vi "Main.vi"() -> ()   [LabVIEW 2018] (continued)
        n137 = Index Array(array=w350, index=2) -> (element=w360:cluster{"X":dbl[], "Y":dbl[]})
        n138 = Index Array(array=w350, index=3) -> (element=w359:cluster{"X":dbl[], "Y":dbl[]})
        n139 = Index Array(array=w350, index=0) -> (element=w362:cluster{"X":dbl[], "Y":dbl[]})
        n140 = Index Array(array=w350, index=1) -> (element=w361:cluster{"X":dbl[], "Y":dbl[]})
        n141 = Unbundle By Name(w359) -> ("Y"=w354:dbl[])
        n142 = Unbundle(w362) -> ("X"=w358:dbl[], "Y"=w357:dbl[])
        n143 = Unbundle By Name(w361) -> ("Y"=w356:dbl[])
        n144 = Unbundle By Name(w360) -> ("Y"=w355:dbl[])
        n145 = Transpose 2D Array(2D array=w371) -> (transposed array=w370:dbl[][])
        n146 = Build Array(w358, w357, w356, w355, w354) -> (w353:dbl[][])
        n147 = Transpose 2D Array(2D array=w353) -> (transposed array=w352:dbl[][])
        n148 = call "Save2CSV.vi"("Time Stamp?"=FALSE, "File Name"=w342, "error in"=w369, "Data Name"="Raw" ("string"), "Data 2D Array"=w370, "Parent Directory"=w364) -> ("error out"=w365:errorcluster)  [unwired: 4 in, 1 out]
        n149 = call "Save2CSV.vi"("Time Stamp?"=FALSE, "File Name"=w342, "error in"=w365, "Data Name"="Phase" ("string"), "Data 2D Array"=w352, "Parent Directory"=w364) -> ("error out"=w351:errorcluster)  [unwired: 4 in, 1 out]
      }
      event "Save #1": Value Change {
        n150 = event-data() -> ()  [unwired: 1 in, 1 out]
        n151 = local read "Wavelength (nm)"() -> (w393:string)
        n152 = local write "Wavelength #1"(w393) -> ()
        "[M/B]#1" <- "[M/B]"
        "Calibrated Bias #1" <- "Calibrated Bias (V)"
        "[O_B] #1" <- "[O_B]"
        "[d13]#1" <- "[d13]"
        "[d24]#1" <- "[d24]"
      }
      event "Load #1": Value Change {
        n153 = event-data() -> ()  [unwired: 1 in, 1 out]
        n154 = local read "[O_B] #1"() -> (w401:dbl)
        n155 = local read "[d13]#1"() -> (w397:dbl)
        n156 = local read "[d24]#1"() -> (w396:dbl)
        n157 = local read "Calibrated Bias #1"() -> (w403:dbl[])
        n158 = local read "[M/B]#1"() -> (w402:dbl)
        n159 = local write "[O_B]"(w401) -> ()
        n160 = local write "Calibrated Bias (V)"(w403) -> ()
        n161 = local write "Wavelength (nm)"("Wavelength #1") -> ()
        n162 = local write "[M/B]"(w402) -> ()
        n163 = local write "[d13]"(w397) -> ()
        n164 = local write "[d24]"(w396) -> ()
      }
      event "Save #2": Value Change {
        n165 = event-data() -> ()  [unwired: 1 in, 1 out]
        n166 = local read "[d13]"() -> (→"[d13]#2":dbl)
        n167 = local read "[O_B]"() -> (→"[O_B]#2":dbl)
        n168 = local read "[d24]"() -> (→"[d24]#2":dbl)
        n169 = local read "Calibrated Bias (V)"() -> (→"Calibrated Bias #2":dbl[])
        n170 = local read "Wavelength (nm)"() -> (w410:string)
        n171 = local read "[M/B]"() -> (→"[M/B]#2":dbl)
        n172 = local write "Wavelength #2"(w410) -> ()
      }
      event "Load #2": Value Change {
        n173 = event-data() -> ()  [unwired: 1 in, 1 out]
        n174 = local read "[O_B]#2"() -> (w421:dbl)
        n175 = local read "[d13]#2"() -> (w417:dbl)
        n176 = local read "Calibrated Bias #2"() -> (w425:dbl[])
        n177 = local read "[d24]#2"() -> (w416:dbl)
        n178 = local read "[M/B]#2"() -> (w424:dbl)
        n179 = local write "[O_B]"(w421) -> ()
        n180 = local write "Wavelength (nm)"("Wavelength #2") -> ()
        n181 = local write "Calibrated Bias (V)"(w425) -> ()
        n182 = local write "[M/B]"(w424) -> ()
        n183 = local write "[d24]"(w416) -> ()
        n184 = local write "[d13]"(w417) -> ()
      }
      event "Save #3": Value Change {
        n185 = event-data() -> ()  [unwired: 1 in, 1 out]
        n186 = local read "[O_B]"() -> (→"[O_B]#3":dbl)
        n187 = local read "[d24]"() -> (→"[d24]#3":dbl)
        n188 = local read "[d13]"() -> (→"[d13]#3":dbl)
        n189 = local read "Calibrated Bias (V)"() -> (→"Calibrated Bias #3":dbl[])
        n190 = local read "Wavelength (nm)"() -> (w430:string)
        n191 = local read "[M/B]"() -> (→"[M/B]#3":dbl)
        n192 = local write "Wavelength #3"(w430) -> ()
      }
      event "Load #3": Value Change {
        n193 = event-data() -> ()  [unwired: 1 in, 1 out]
        n194 = local read "[O_B]#3"() -> (w441:dbl)
        n195 = local read "[d13]#3"() -> (w437:dbl)
        n196 = local read "[d24]#3"() -> (w436:dbl)
        n197 = local read "Calibrated Bias #3"() -> (w443:dbl[])
        n198 = local read "[M/B]#3"() -> (w442:dbl)
        n199 = local write "[O_B]"(w441) -> ()
        n200 = local write "Wavelength (nm)"("Wavelength #3") -> ()
        n201 = local write "Calibrated Bias (V)"(w443) -> ()
        n202 = local write "[M/B]"(w442) -> ()
        n203 = local write "[d13]"(w437) -> ()
        n204 = local write "[d24]"(w436) -> ()
      }
      event "Save #4": Value Change {
        n205 = event-data() -> ()  [unwired: 1 in, 1 out]
        n206 = local read "[d13]"() -> (→"[d13]#4":dbl)
        n207 = local read "[d24]"() -> (→"[d24]#4":dbl)
        n208 = local read "[O_B]"() -> (→"[O_B]#4":dbl)
        n209 = local read "Calibrated Bias (V)"() -> (→"Calibrated Bias #4":dbl[])
        n210 = local read "Wavelength (nm)"() -> (w450:string)
        n211 = local read "[M/B]"() -> (→"[M/B]#4":dbl)
        n212 = local write "Wavelength #4"(w450) -> ()
      }
      event "Load #4": Value Change {
        n213 = event-data() -> ()  [unwired: 1 in, 1 out]
        n214 = local read "[O_B]#4"() -> (w461:dbl)
        n215 = local read "[d13]#4"() -> (w457:dbl)
        n216 = local read "Calibrated Bias #4"() -> (w463:dbl[])
        n217 = local read "[d24]#4"() -> (w456:dbl)
        n218 = local read "[M/B]#4"() -> (w462:dbl)
        n219 = local write "[O_B]"(w461) -> ()
        n220 = local write "Wavelength (nm)"("Wavelength #4") -> ()
        n221 = local write "Calibrated Bias (V)"(w463) -> ()
        n222 = local write "[M/B]"(w462) -> ()
        n223 = local write "[d13]"(w457) -> ()
        n224 = local write "[d24]"(w456) -> ()
      }
      event "Fast Scan": Value Change {
        # "Repeat for Fast Scan"
        n225 = event-data() -> ()  [unwired: 1 in, 1 out]
        n226 = flat-sequence {
          tunnel: w482 -> [w489]
          tunnel: [w489] -> w478
          tunnel: [w488] -> w477
          tunnel: [w487] -> w476
          tunnel: w480 -> [w487]
          tunnel: [w486] -> w475
          tunnel: w479 -> [w486]
          tunnel: w474 -> [w484]
          tunnel: [w483] -> w473
          tunnel: w478 -> [w518]
          tunnel: [w518] -> w470
          tunnel: w477 -> [w517]
          tunnel: [w517] -> w469
          tunnel: w476 -> [w513]
          tunnel: w475 -> [w500]
          tunnel: [w510] -> w468
          tunnel: w473 -> [w509]
          tunnel: [w498] -> w466
          tunnel: [w546] -> w472
          tunnel: [w547] -> w481
          tunnel: w470 -> [w547]
          tunnel: w468 -> [w543]
          tunnel: w469 -> [w537]
          tunnel: w466 -> [w530]
          frame #0 {
            n227 = local read "Shutter"() -> (w485:bool)
            n228 = case shown="False" w485 {
              tunnel: w484 -> [w493 w495]
              tunnel: [w492 w495] -> w483
              frame False {
                n229 = local read "Shutter Line"() -> (w490:tag)
                n230 = call "ShutterControl.vi"("error in"=w493, "Shutter Line"=w490, "Shutter"=TRUE) -> ("error out"=w492:errorcluster, "Status Indicator"=w491:bool)  [unwired: 7 in]
                n231 = local write "Shutter"(w491) -> ()
              }
              frame True {
              }
            }
            n232 = Tick Count (ms)() -> (millisecond timer value=w488:u32)
          }
          frame #1 {
            w503 = T13."Fast Scan" ("Main Tab")
            n233 = local read "AOStartTrigger"() -> (w496:tag)
            n234 = local read "AIStartTrigger"() -> (w497:tag)
            n235 = call "DAQInit.vi"("AOStartTrigger"=w496, "AIStartTrigger"=w497, "Scan/Meas Parameters"="Fast Scan Parameters", "error in"=w509, "Functions"=w503, "Global Parameters"=w500, "DAQ Channels"=w513) -> ("error out"=w511:errorcluster, "Expected Time (s)"=→"Expected Frame Time (s)":dbl, "Tasks Out"=w515:T14)  [unwired: 2 in]
            n236 = call "ScanXY.vi"("Scan/Meas Parameters"="Fast Scan Parameters") -> ("XYcoordinates"=w504:dbl[][])  [unwired: 10 in]
            n237 = Unbundle By Name("Fast Scan Parameters") -> ("Pixel Size"=w508:dbl)
            n238 = case shown="True" "Single Pixel?" {
              tunnel: [w519 w520] -> w505
              tunnel: w504 -> [w519 w521]
              frame False {
              }
              frame True {
                n239 = Multiply(x=w521, y=0.0) -> (x*y=w520:dbl[][])
              }
            }
            n240 = To Long Integer(number=w508) -> (32bit integer=w507:i32)
            n241 = call "ImageFrame.vi"("Tasks In"=w515, "Functions"=w503, "error in"=w511, "XYcoordinates"=w505) -> ("Tasks Out"=w512:T14, "DC AI Channel Date"=w501:dbl[], "error out"=w514:errorcluster)  [unwired: 7 in, 2 out]
            n242 = call "Analysis.vi"("Functions"=w503, "Scan/Meas Parameters"="Fast Scan Parameters", "Global Parameters"=w500, "DC AI Channel Data"=w501) -> ("AI DC Data"=w498:dbl[])  [unwired: 2 in, 5 out]
            n243 = Reshape Array(w498, w507, w507) -> (→"Fast Scan Intensity Image":dbl[][])
            n244 = call "DAQClose.vi"("error in"=w514, "Functions"=w503, "Tasks In"=w512, "DAQ Channels"=w513) -> ("error out"=w510:errorcluster)  [unwired: 7 in]
          }
          frame #2 {
            n245 = local read "Simple Max Search"() -> (w533:bool)
            n246 = local read "Shutter Line"() -> (w523:tag)
            n247 = local read "Export Z Calibration"() -> (w524:bool)
            n248 = Tick Count (ms)() -> (millisecond timer value=w538:u32)
            n249 = call "ShutterControl.vi"("error in"=w543, "Shutter Line"=w523, "Shutter"=FALSE) -> ("error out"=w542:errorcluster, "Status Indicator"=w544:bool)  [unwired: 7 in]
            n250 = local read "Quadratic Search"() -> (w526:bool)
            n251 = local write "Shutter"(w544) -> ()
            n252 = call <vilib>:"Std Deviation and Variance.vi"("X"=w530) -> ("mean"=w525:dbl, "variance"=w531:dbl)  [unwired: 1 in, 1 out]
            "Mean Pixel Value" <- w525
            n253 = Subtract(x=w538, y=w537) -> (x-y=w540:u32)
            n254 = Square(x=w525) -> (x^2=w532:dbl)
            n255 = local read "SPGD"() -> (w534:bool)
            n256 = To Double Precision Float(number=w540) -> (double precision float=w541:dbl)
            n257 = Divide(x=w531, y=w532) -> (x/y=w527:dbl)
            "Normalized Variance" <- w527
            n258 = Divide(x=w541, y=1000.0) -> (x/y=→"Actual Scan Time (s)":dbl)
            n259 = Compound Arithmetic op=OR(w526, w534, w533, w524) -> (w535:bool)
            n260 = case shown="False" w535 {
              tunnel: [w563 w570] -> w546
              tunnel: w542 -> [w561 w570]
              frame False {
                n261 = local read "Fast Scan Progress"() -> (w557:dbl)
                n262 = Reciprocal(x="Fast Scan Frames") -> (1/x=w558:dbl)
                n263 = Multiply(x=100.0, y=w558) -> (x*y=w560:dbl)
                n264 = Add(x=w557, y=w560) -> (x+y=w553:dbl)
                "Fast Scan Progress" <- w553
                n265 = Greater Or Equal?(x=w553, y=100.0) -> (x >= y?=w554:bool)
                n266 = Compound Arithmetic op=OR(w554, "Stop Fast Scan") -> (w562:bool)
                n267 = case shown="True" w562 {
                  tunnel: w561 -> [w566 w567]
                  tunnel: [w565 w567] -> w563
                  frame False {
                    # "Continue Fast Scan"
                    n268 = property on="Fast Scan" class="Bool (strict)"(error in=w566, "Val(Sgnl)"=TRUE ("Value (Signaling)")) -> (error out=w565:errorcluster)  [unwired: 1 in, 1 out]
                  }
                  frame True {
                    w569 = FALSE ("Fast Scan")
                    # "Fast Scan Stops"
                    n269 = local write "Fast Scan Progress"(0.0 ("Fast Scan Progress")) -> ()
                    n270 = local write "Fast Scan"(w569) -> ()
                    n271 = local write "Stop Fast Scan"(w569) -> ()
                  }
                }
              }
              frame True {
              }
            }
            n272 = case shown="\"Mean Pixel Value\", Default" "Optimization Metric" {
              tunnel: [w548 w549 w550] -> w528
              tunnel: w525 -> [w548 _ w551]
              tunnel: w527 -> [_ w549 _]
              frame "Mean Pixel Value", Default {
              }
              frame "Normalized Variance" {
              }
              frame "Mean Squared Pixel Value" {
                n273 = Square Root(x=w551) -> (sqrt(x)=w550:dbl)
              }
            }
            "Metric Value" <- w528
          }
        }
      }
      event "Relax DM": Value Change {
        n274 = event-data() -> ()  [unwired: 1 in, 1 out]
        n275 = local read "Use DM?"() -> (w571:bool)
        n276 = case shown="True" w571 {
          tunnel: [w579 w583] -> w576
          tunnel: [w578 w582] -> w575
          tunnel: w573 -> [w579 w581]
          tunnel: w572 -> [w578 w580]
          frame False {
          }
          frame True {
            w591 = u32 0 items=["Mirror", "Arms", "Mirror + Arms"] ("Device Part (Mirror)")
            # "First Step"
            n277 = call "TLDFMX Relax.vi"("Reload (1)"=TRUE, "error in (no error)"=w580, "Is First Step (0)"=TRUE, "Device Part (Mirror)"=w591, "instrument handle"=w581) -> ("error out"=w587:errorcluster, "Relax Pattern Mirror (0)"=w586:dbl[], "instrument handle out"=w588:refnum<visa-resource-name>)  [unwired: 2 in, 2 out]
            n278 = call "TLDFM Set Segment Voltages.vi"("error in (no error)"=w587, "Segment Voltages"=w586, "instrument handle"=w588) -> ("error out"=w584:errorcluster, "instrument handle out"=w585:refnum<visa-resource-name>)  [unwired: 7 in]
            n279 = while {
              tunnel: w585 -> [w597]
              tunnel: w584 -> [w596]
              tunnel: [w593] -> w583
              tunnel: [w592] -> w582
              stop <- w594 stop-if-true
              w598 = u32 0 items=["Mirror", "Arms", "Mirror + Arms"] ("Device Part (Mirror)")
              # "Loop Until Remaining Relax Steps Are 0"
              n280 = call "TLDFMX Relax.vi"("Reload (1)"=TRUE, "error in (no error)"=w596, "Is First Step (0)"=FALSE, "Device Part (Mirror)"=w598, "instrument handle"=w597) -> ("error out"=w602:errorcluster, "Relax Pattern Mirror (0)"=w603:dbl[], "instrument handle out"=w601:refnum<visa-resource-name>, "Remaining Steps"=w595:i32)  [unwired: 2 in, 1 out]
              n281 = Less Or Equal To 0?(x=w595) -> (x <= 0?=w594:bool)
              n282 = call "TLDFM Set Segment Voltages.vi"("error in (no error)"=w602, "Segment Voltages"=w603, "instrument handle"=w601) -> ("error out"=w592:errorcluster, "instrument handle out"=w593:refnum<visa-resource-name>)  [unwired: 7 in]
            }
          }
        }
      }
      event "Reset Zernike": Value Change {
        n283 = event-data() -> ()  [unwired: 1 in, 1 out]
        n284 = local read "Use DM?"() -> (w604:bool)
        n285 = local write "Zernike Array"(dbl[] [0.0, 0.0, 0.0, 0.0, 0.0, 0.0, 0.0, 0.0, 0.0, 0.0, 0.0, 0.0] ("Zernike Array")) -> ()
        n286 = case shown="False" w604 {
          tunnel: w608 -> [w612 w616]
          tunnel: w607 -> [w611 w615]
          tunnel: [w612 w614] -> w606
          tunnel: [w611 w613] -> w605
          frame False {
          }
          frame True {
            n287 = call "TLDFMX Reset.vi"("error in (no error)"=w615, "instrument handle"=w616) -> ("error out"=w613:errorcluster, "instrument handle out"=w614:refnum<visa-resource-name>)  [unwired: 8 in]
          }
        }
      }
      event "Zernike Array", "Apply Zernike": Value Change {
        n288 = event-data() -> ()  [unwired: 1 in, 1 out]
        n289 = local read "Use DM?"() -> (w617:bool)
        n290 = case shown="True" w617 {
          tunnel: w623 -> [w624 w637]
          tunnel: w622 -> [w625 w635]
          tunnel: [w624 w631] -> w621
          tunnel: [w625 w630] -> w619
          frame False {
          }
          frame True {
            n291 = local read "Zernike Enable"() -> (w629:bool[])
            n292 = Boolean To (0,1)(Boolean=w629) -> (0, 1=w628:i16[])
            n293 = Multiply(x="Zernike Array", y=w628) -> (x*y=w626:dbl[])
            n294 = call "TLDFMX Calculate Zernike Pattern.vi"("error in (no error)"=w637, "Zernike Amplitudes"=w626, "Zernikes"=u32 4294967295, "instrument handle"=w635) -> ("error out"=w632:errorcluster, "Mirror Pattern"=w633:dbl[], "instrument handle out"=w634:refnum<visa-resource-name>)  [unwired: 5 in]
            n295 = call "TLDFM Set Segment Voltages.vi"("error in (no error)"=w632, "Segment Voltages"=w633, "instrument handle"=w634) -> ("error out"=w631:errorcluster, "instrument handle out"=w630:refnum<visa-resource-name>)  [unwired: 7 in]
          }
        }
      }
      event "Save Zernike": Value Change {
        w655 = "DM" ("section")
        n296 = event-data() -> ()  [unwired: 1 in, 1 out]
        n297 = Current VI's Path() -> (path=w639:path)
        n298 = Strip Path(path=w639) -> (stripped path=w638:path)  [unwired: 1 out]
        n299 = Build Path(base path=w638, name or relative path=path "config.ini" ("default name")) -> (appended path=w665:path)
        n300 = local read "Zernike Array"() -> (w649:dbl[])
        n301 = call <vilib>:"Open Config Data.vi"("error in (no error)"=w664, "create file if necessary (T)"=TRUE, "configuration file path"=w665) -> ("error out"=w663:errorcluster, "refnum"=w661:T15)  [unwired: 6 in, 1 out]
        n302 = Array To Spreadsheet String(delimiter (Tab)=",", array=w649, 3:"%#g" ("format string")) -> (spreadsheet string=w653:string)
        n303 = Search and Replace String(input string=w653, search string="\r\n") -> (result string=w648:string)  [unwired: 6 in, 3 out]
        n304 = call-poly <vilib>:"Write Key.vi"("section"=w655, "error in (no error)"=w663, "value"=w648, "key"="Zernike Array", "refnum"=w661) -> ("error out"=w657:errorcluster, "refnum out"=w659:T15)  [unwired: 4 in, 1 out]
        n305 = local read "Zernike Enable"() -> (w642:bool[])
        n306 = for {
          tunnel: w642 -> [w670] mode=indexing
          tunnel: [w669] -> w643 mode=indexing
          n307 = Select(t="TRUE", s=w670, f="FALSE") -> (s? t:f=w669:string)
        }
        n308 = Array To Spreadsheet String(delimiter (Tab)=",", array=w643, 3:"%s" ("format string")) -> (spreadsheet string=w647:string)
        n309 = Search and Replace String(input string=w647, search string="\r\n") -> (result string=w641:string)  [unwired: 6 in, 3 out]
        n310 = call-poly <vilib>:"Write Key.vi"("section"=w655, "error in (no error)"=w657, "value"=w641, "key"="Zernike Enable", "refnum"=w659) -> ("error out"=w656:errorcluster, "refnum out"=w658:T15)  [unwired: 4 in, 1 out]
        n311 = call <vilib>:"Close Config Data.vi"("error in (no error)"=w656, "refnum"=w658) -> ("error out"=w662:errorcluster)  [unwired: 8 in, 1 out]
      }
      event "Load Zernike": Value Change {
        n312 = event-data() -> ()  [unwired: 1 in, 1 out]
        n313 = Current VI's Path() -> (path=w680:path)
        n314 = Strip Path(path=w680) -> (stripped path=w679:path)  [unwired: 1 out]
        n315 = Build Path(base path=w679, name or relative path=path "config.ini" ("default name")) -> (appended path=w677:path)
        n316 = call <vilib>:"Check if File or Folder Exists.vi"("error in (no error)"=w676, "path"=w677) -> ("error out"=w675:errorcluster, "file or folder exists?"=w673:bool, "dup path"=w674:path)  [unwired: 7 in]
        n317 = case shown="True" w673 {
          tunnel: [w684 w708] -> w678
          tunnel: w675 -> [w684 w686]
          tunnel: w674 -> [_ w685]
          frame False {
          }
          frame True {
            w688 = "DM" ("section")
            n318 = call <vilib>:"Open Config Data.vi"("error in (no error)"=w686, "create file if necessary (T)"=FALSE, "configuration file path"=w685) -> ("error out"=w701:errorcluster, "refnum"=w702:T15)  [unwired: 6 in, 1 out]
            n319 = call-poly <vilib>:"Read Key.vi"("section"=w688, "error in (no error)"=w701, "key"="Zernike Array", "refnum"=w702) -> ("error out"=w693:errorcluster, "value"=w704:string, "refnum out"=w691:T15)  [unwired: 4 in, 1 out]
            n320 = Spreadsheet String To Array(delimiter (Tab)=",", format string="%s", spreadsheet string=w704, array type (2D Dbl)=dbl[] []) -> (array=w700:dbl[])
            n321 = local write "Zernike Array"(w700) -> ()
            n322 = call-poly <vilib>:"Read Key.vi"("section"=w688, "error in (no error)"=w693, "key"="Zernike Enable", "refnum"=w691) -> ("error out"=w692:errorcluster, "value"=w696:string, "refnum out"=w690:T15)  [unwired: 4 in, 1 out]
            n323 = Spreadsheet String To Array(delimiter (Tab)=",", format string="%s", spreadsheet string=w696, array type (2D Dbl)=string[] []) -> (array=w694:string[])
            n324 = for {
              tunnel: "TRUE" -> [w712]
              tunnel: w694 -> [w711] mode=indexing
              tunnel: [w710] -> w687 mode=indexing
              n325 = Equal?(x=w711, y=w712) -> (x = y?=w710:bool)
            }
            n326 = local write "Zernike Enable"(w687) -> ()
            n327 = call <vilib>:"Close Config Data.vi"("error in (no error)"=w692, "refnum"=w690) -> ("error out"=w708:errorcluster)  [unwired: 8 in, 1 out]
          }
        }
      }
      event "Quadratic Search": Value Change {
        n328 = event-data() -> ()  [unwired: 1 in, 1 out]
        n329 = while {
          tunnel: [w814] -> w720
          tunnel: [w816] -> w724
          stop <- w817 stop-if-true
          n330 = local read "Zernike Enable"() -> (w815:bool[])
          n331 = local read "Current Z Idx"() -> (w820:i32)
          n332 = Index Array(array=w815, index=w820) -> (element=w821:bool)
          n333 = Array Size(array=w815) -> (size(s)=w819:i32)
          n334 = case shown="True" w821 {
            tunnel: w820 -> [w825 w827]
            tunnel: [w824 w827] -> w814
            tunnel: [FALSE ("2D Time-Lapse Measure") TRUE ("2D Time-Lapse Measure")] -> w818
            frame False {
              n335 = local write "Z Direction"(TRUE ("Zernike Dir")) -> ()
              n336 = Increment(x=w825) -> (x+1=w824:i32)
            }
            frame True {
            }
          }
          n337 = Greater?(x=w814, y=w819) -> (0:w816:bool)
          n338 = local write "Current Z Idx"(w814) -> ()
          n339 = Compound Arithmetic op=OR(w818, w816) -> (w817:bool)
        }
        n340 = local read "Current Iteration"() -> (w713:sgl)
        n341 = local read "Quadratic Calc"() -> (w716:bool)
        n342 = case shown="False" w716 {
          tunnel: w715 -> [w727 w731]
          tunnel: [w727 w731] -> w714
          tunnel: w713 -> [w726 _]
          frame False {
            n343 = Equal To 0?(x=w726) -> (x = 0?=w725:bool)
            n344 = case shown="True" w725 {
              frame False {
              }
              frame True {
                n345 = local read "Zernike Array"() -> (w728:dbl[])
                n346 = local write "Optimal Z Idx"(0 ("Optimal Z Idx")) -> ()
                n347 = local write "Optimal Zernike"(w728) -> ()
              }
            }
          }
          frame True {
            n348 = local read "Bias Amplitude"() -> (w740:dbl)
            n349 = local read "Optimal Zernike"() -> (w734:dbl[])
            n350 = local read "Initial Metric"() -> (w742:dbl)
            n351 = local read "Metric Value"() -> (w741:dbl)
            n352 = local read "Last Metric"() -> (w743:dbl)
            n353 = local read "Optimal Z Idx"() -> (w730:i32)
            n354 = call "QuadraticOptimization.vi"("Bias Amplitude"=w740, "Neg Metric"=w741, "Initial Metric"=w742, "Pos Metric"=w743) -> ("Opt Variable (compared to 0)"=w732:dbl)  [unwired: 7 in]
            n355 = Index Array(array=w734, index=w730) -> (element=w736:dbl)
            n356 = Add(x=w736, y=w732) -> (x+y=w737:dbl)
            n357 = In Range and Coerce(upper limit=1.0 ("y"), x=w737, lower limit=-1.0 ("y")) -> (coerced(x)=w735:dbl)  [unwired: 1 out]
            n358 = Replace Array Subset(array=w734, new element=w735, index=w730) -> (→"Optimal Zernike":dbl[])
          }
        }
        n359 = local read "Stop AO Algorithm"() -> (w723:bool)
        n360 = Compound Arithmetic op=OR(w724, w723) -> (w722:bool)
        n361 = case shown="False" w722 {
          tunnel: w714 -> [w755 w803]
          tunnel: [w750 w802] -> w721
          tunnel: w718 -> [w756 w800]
          tunnel: [w757 w801] -> w717
          tunnel: w713 -> [w747 _]
          tunnel: w720 -> [w752 _]
          frame False {
            w749 = TRUE ("Value (Signaling)")
            n362 = Equal To 0?(x=w747) -> (x = 0?=w753:bool)
            n363 = case shown="False" w753 {
              tunnel: [w776 w793] -> w748
              tunnel: [w778 w794] -> w744
              tunnel: w752 -> [w764 _]
              frame False {
                n364 = local read "Initial Zernike"() -> (w765:dbl[])
                n365 = local read "Z Direction"() -> (w775:bool)
                n366 = case shown="False" w775 {
                  tunnel: "Bias Amplitude" -> [w786 w791]
                  tunnel: [w785 w791] -> w773
                  tunnel: [FALSE ("Zernike Dir") TRUE ("Zernike Dir")] -> w768
                  tunnel: w764 -> [w782 _]
                  frame False {
                    # "Negative Bias"
                    n367 = Multiply(x=w786, y=-1.0) -> (x*y=w785:dbl)
                    "Quadratic Calc" <- TRUE ("Quadratic Calc")
                    "Optimal Z Idx" <- w782
                  }
                  frame True {
                    # "Positive Bias"
                    n368 = local write "Quadratic Calc"(FALSE ("Zernike Dir")) -> ()
                    n369 = local write "Z Direction"(FALSE ("Zernike Dir")) -> ()
                  }
                }
                n370 = Index Array(array=w765, index=w764) -> (element=w777:dbl)
                n371 = Add(x=w777, y=w773) -> (x+y=w770:dbl)
                n372 = In Range and Coerce(upper limit=1.0 ("y"), x=w770, lower limit=-1.0 ("y")) -> (coerced(x)=w769:dbl, In Range?=w767:bool)
                n373 = Compound Arithmetic op=AND(w767, w768) -> (w766:bool)
                n374 = case shown="False" w766 {
                  tunnel: w764 -> [w780 _]
                  frame False {
                    n375 = Increment(x=w780) -> (x+1=w781:i32)
                    n376 = local write "Z Direction"(TRUE ("Zernike Dir")) -> ()
                    n377 = local write "Current Z Idx"(w781) -> ()
                  }
                  frame True {
                  }
                }
                n378 = local read "Metric Value"() -> (w778:dbl)
                n379 = Replace Array Subset(array=w765, new element=w769, index=w764) -> (w776:dbl[])
              }
              frame True {
                n380 = local read "Zernike Array"() -> (w793:dbl[])
                "Initial Zernike" <- w793
                n381 = local read "Last Metric"() -> (w794:dbl)
                n382 = local write "Quadratic Calc"(FALSE ("Zernike Dir")) -> ()
              }
            }
            n383 = Increment(x=w747) -> (x+1=w754:sgl)
            n384 = local write "Current Iteration"(w754) -> ()
            n385 = call "TLDFMX Calculate Zernike Pattern.vi"("error in (no error)"=w755, "Zernike Amplitudes"=w748, "Zernikes"=u32 4294967295, "instrument handle"=w756) -> ("error out"=w759:errorcluster, "Mirror Pattern"=w760:dbl[], "instrument handle out"=w761:refnum<visa-resource-name>)  [unwired: 5 in]
            n386 = call "TLDFM Set Segment Voltages.vi"("error in (no error)"=w759, "Segment Voltages"=w760, "instrument handle"=w761) -> ("error out"=w758:errorcluster, "instrument handle out"=w757:refnum<visa-resource-name>)  [unwired: 7 in]
            n387 = Equal?(x=w747, y=sgl 1.0) -> (x = y?=w745:bool)
            n388 = property on="Fast Scan" class="Bool (strict)"(error in=w758, "Val(Sgnl)"=w749) -> (error out=w751:errorcluster)  [unwired: 1 in, 1 out]
            n389 = case shown="True" w745 {
              tunnel: w744 -> [_ w763]
              frame False {
              }
              frame True {
                "Initial Metric" <- w763
              }
            }
            n390 = local write "Zernike Array"(w748) -> ()
            n391 = property on="Quadratic Search" class="Bool (strict)"(error in=w751, "Val(Sgnl)"=w749) -> (error out=w750:errorcluster)  [unwired: 1 in, 1 out]
            n392 = local write "Last Metric"(w744) -> ()
          }
          frame True {
            w813 = FALSE ("2D Time-Lapse Measure")
            n393 = local read "Zernike Enable"() -> (w799:bool[])
            n394 = local read "Optimal Zernike"() -> (w797:dbl[])
            n395 = Boolean To (0,1)(Boolean=w799) -> (0, 1=w798:i16[])
            n396 = Multiply(x=w797, y=w798) -> (x*y=w796:dbl[])
            n397 = call "TLDFMX Calculate Zernike Pattern.vi"("error in (no error)"=w803, "Zernike Amplitudes"=w796, "Zernikes"=u32 4294967295, "instrument handle"=w800) -> ("error out"=w804:errorcluster, "Mirror Pattern"=w805:dbl[], "instrument handle out"=w806:refnum<visa-resource-name>)  [unwired: 5 in]
            n398 = local write "Zernike Array"(w797) -> ()
            n399 = call "TLDFM Set Segment Voltages.vi"("error in (no error)"=w804, "Segment Voltages"=w805, "instrument handle"=w806) -> ("error out"=w802:errorcluster, "instrument handle out"=w801:refnum<visa-resource-name>)  [unwired: 7 in]
            n400 = local write "Optimal Z Idx"(0 ("Optimal Z Idx")) -> ()
            n401 = local write "Quadratic Calc"(FALSE ("Zernike Dir")) -> ()
            n402 = local write "Current Iteration"(sgl 0.0 ("Current Step")) -> ()
            n403 = local write "Quadratic Search"(w813) -> ()
            n404 = local write "Z Direction"(TRUE ("Zernike Dir")) -> ()
            n405 = local write "Fast Scan Progress"(0.0 ("Fast Scan Progress")) -> ()
            n406 = local write "Current Z Idx"(0 ("Curr Zernike Idx")) -> ()
            n407 = local write "Fast Scan"(w813) -> ()
            n408 = local write "Stop Fast Scan"(w813) -> ()
            n409 = local write "Stop AO Algorithm"(w813) -> ()
          }
        }
      }
      event "Simple Max Search": Value Change {
        n410 = event-data() -> ()  [unwired: 1 in, 1 out]
        n411 = while {
          tunnel: [w838] -> w828
          tunnel: [w840] -> w830
          stop <- w841 stop-if-true
          n412 = local read "Zernike Enable"() -> (w839:bool[])
          n413 = local read "Current Z Idx"() -> (w844:i32)
          n414 = Index Array(array=w839, index=w844) -> (element=w845:bool)
          n415 = Array Size(array=w839) -> (size(s)=w843:i32)
          n416 = case shown="False" w845 {
            tunnel: w844 -> [w849 w851]
            tunnel: [w848 w851] -> w838
            tunnel: [FALSE ("2D Time-Lapse Measure") TRUE ("2D Time-Lapse Measure")] -> w842
            frame False {
              n417 = local write "Z Direction"(TRUE ("Zernike Dir")) -> ()
              n418 = Increment(x=w849) -> (x+1=w848:i32)
            }
            frame True {
            }
          }
          n419 = Greater?(x=w838, y=w843) -> (0:w840:bool)
          n420 = local write "Current Z Idx"(w838) -> ()
          n421 = Compound Arithmetic op=OR(w842, w840) -> (w841:bool)
        }
        n422 = local read "Stop AO Algorithm"() -> (w832:bool)
        n423 = local read "Current Iteration"() -> (w829:sgl)
        n424 = Compound Arithmetic op=OR(w830, w832) -> (w831:bool)
        n425 = case shown="False" w831 {
          tunnel: w836 -> [w852 w909]
          tunnel: w835 -> [w853 w910]
          tunnel: [w867 w910] -> w834
          tunnel: [w864 w909] -> w833
          tunnel: w829 -> [w856 _]
          tunnel: w828 -> [w857 _]
          frame False {
            w863 = TRUE ("Value (Signaling)")
            n426 = Equal To 0?(x=w856) -> (x = 0?=w862:bool)
            n427 = Increment(x=w856) -> (x+1=w855:sgl)
            n428 = case shown="True" w862 {
              tunnel: [w879 w905] -> w859
              tunnel: w857 -> [w874 _]
              tunnel: [w872 w904] -> w854
              frame False {
                n429 = local read "Metric Value"() -> (w872:dbl)
                n430 = local read "Zernike Array"() -> (w881:dbl[])
                n431 = local read "Last Metric"() -> (w873:dbl)
                n432 = local read "Z Direction"() -> (w875:bool)
                n433 = Greater?(x=w872, y=w873) -> (0:w878:bool)
                n434 = Index Array(array=w881, index=w874) -> (element=w882:dbl)
                n435 = case shown="True" w875 {
                  tunnel: w878 -> [w886 w897]
                  tunnel: "Step Size" -> [w885 w896]
                  tunnel: [w884 w895] -> w876
                  tunnel: w874 -> [w883 _]
                  frame False {
                    # "Decreasing Zernike Coefficient"
                    n436 = case shown="True" w886 {
                      tunnel: w885 -> [w890 w892]
                      tunnel: [w890 w891] -> w884
                      tunnel: w883 -> [w888 _]
                      frame False {
                        n437 = Increment(x=w888) -> (x+1=w889:i32)
                        n438 = local write "Z Direction"(TRUE ("Zernike Dir")) -> ()
                        n439 = local write "Current Z Idx"(w889) -> ()
                      }
                      frame True {
                        n440 = local write "Z Direction"(FALSE ("Zernike Dir")) -> ()
                        n441 = Multiply(x=w892, y=-1.0) -> (x*y=w891:dbl)
                      }
                    }
                  }
                  frame True {
                    # "Increasing Zernike Coefficient"
                    n442 = case shown="False" w897 {
                      tunnel: w896 -> [w901 w903]
                      tunnel: [w900 w903] -> w895
                      frame False {
                        n443 = local write "Z Direction"(FALSE ("Zernike Dir")) -> ()
                        n444 = Multiply(x=w901, y=-1.0) -> (x*y=w900:dbl)
                      }
                      frame True {
                        "Z Direction" <- TRUE ("Zernike Dir")
                      }
                    }
                  }
                }
                n445 = Add(x=w882, y=w876) -> (x+y=w880:dbl)
                n446 = Replace Array Subset(array=w881, new element=w880, index=w874) -> (w879:dbl[])
              }
              frame True {
                n447 = local read "Zernike Array"() -> (w905:dbl[])
                n448 = local read "Last Metric"() -> (w904:dbl)
              }
            }
            "Last Metric" <- w854
            n449 = local write "Current Iteration"(w855) -> ()
            n450 = In Range and Coerce(upper limit=1.0 ("y"), x=w859, lower limit=-1.0 ("y")) -> (coerced(x)=w858:dbl[])  [unwired: 1 out]
            n451 = call "TLDFMX Calculate Zernike Pattern.vi"("error in (no error)"=w852, "Zernike Amplitudes"=w858, "Zernikes"=u32 4294967295, "instrument handle"=w853) -> ("error out"=w868:errorcluster, "Mirror Pattern"=w869:dbl[], "instrument handle out"=w870:refnum<visa-resource-name>)  [unwired: 5 in]
            n452 = call "TLDFM Set Segment Voltages.vi"("error in (no error)"=w868, "Segment Voltages"=w869, "instrument handle"=w870) -> ("error out"=w866:errorcluster, "instrument handle out"=w867:refnum<visa-resource-name>)  [unwired: 7 in]
            n453 = property on="Fast Scan" class="Bool (strict)"(error in=w866, "Val(Sgnl)"=w863) -> (error out=w865:errorcluster)  [unwired: 1 in, 1 out]
            n454 = local write "Zernike Array"(w858) -> ()
            n455 = property on="Simple Max Search" class="Bool (strict)"(error in=w865, "Val(Sgnl)"=w863) -> (error out=w864:errorcluster)  [unwired: 1 in, 1 out]
          }
          frame True {
            w911 = FALSE ("2D Time-Lapse Measure")
            n456 = local write "Z Direction"(TRUE ("Zernike Dir")) -> ()
            n457 = local write "Simple Max Search"(w911) -> ()
            n458 = local write "Fast Scan Progress"(0.0 ("Fast Scan Progress")) -> ()
            n459 = local write "Current Iteration"(sgl 0.0 ("Current Step")) -> ()
            n460 = local write "Fast Scan"(w911) -> ()
            n461 = local write "Stop Fast Scan"(w911) -> ()
            n462 = local write "Stop AO Algorithm"(w911) -> ()
            "Current Z Idx" <- 0 ("Curr Zernike Idx")
          }
        }
      }
      event "SPGD": Value Change {
        n463 = event-data() -> ()  [unwired: 1 in, 1 out]
        n464 = local read "Current Iteration"() -> (w923:sgl)
        n465 = To Single Precision Float(number="Total Iteration") -> (single precision float=w915:sgl)
        n466 = Greater Or Equal?(x=w923, y=w915) -> (x >= y?=w921:bool)
        n467 = Compound Arithmetic op=OR(w921, "Stop AO Algorithm") -> (w922:bool)
        n468 = case shown="False" w922 {
          tunnel: w923 -> [w932 _]
          tunnel: w919 -> [w926 w983]
          tunnel: [w935 w983] -> w914
          tunnel: w918 -> [w927 w982]
          tunnel: [w944 w982] -> w917
          frame False {
            w937 = TRUE ("Value (Signaling)")
            n469 = Equal To 0?(x=w932) -> (x = 0?=w939:bool)
            n470 = Quotient & Remainder(x=w932, y=sgl 1.0) -> (x-y*floor(x/y)=w951:sgl)  [unwired: 1 out]
            n471 = local read "Metric Value"() -> (w925:dbl)
            n472 = local read "Zernike Array"() -> (w943:dbl[])
            n473 = Equal?(x=w951, y=sgl 0.5) -> (x = y?=w949:bool)
            n474 = Add(x=w932, y=sgl 0.5) -> (x+y=→"Current Iteration":sgl)
            n475 = case shown="True" w949 {
              tunnel: [w955 w968] -> w940
              tunnel: w943 -> [_ w967]
              tunnel: w939 -> [w954 _]
              tunnel: w925 -> [w953 w966]
              frame False {
                # "Before First Sub-Step"
                n476 = case shown="False" w954 {
                  tunnel: [w958 w965] -> w955
                  tunnel: w953 -> [w962 _]
                  frame False {
                    n477 = local read "Sigma"() -> (w963:dbl[])
                    n478 = local read "Last Metric"() -> (w956:dbl)
                    n479 = local read "Last Zernike"() -> (w957:dbl[])
                    n480 = Multiply(x="Learning Rate", y=w963) -> (x*y=w961:dbl[])
                    n481 = Subtract(x=w962, y=w956) -> (x-y=w960:dbl)
                    n482 = Multiply(x=w961, y=w960) -> (x*y=w959:dbl[])
                    n483 = Subtract(x=w957, y=w959) -> (x-y=w958:dbl[])
                  }
                  frame True {
                    n484 = local read "Zernike Array"() -> (w965:dbl[])
                  }
                }
              }
              frame True {
                # "Before Second Sub-Step"
                n485 = local write "Last Metric"(w966) -> ()
                n486 = Array Size(array=w967) -> (size(s)=w970:i32)
                n487 = for {
                  N: w970 -> [_]
                  tunnel: [w971] -> w969 mode=indexing
                  # "4 possibilities, [0, 4)"
                  n488 = Random Number (0-1)() -> (number: 0 to 1=w975:dbl)
                  n489 = Multiply(x=w975, y=4.0) -> (x*y=w973:dbl)
                  n490 = Round Toward -Infinity(1:w973) -> (0:w972:dbl)
                  n491 = case shown="3" w972 {
                    tunnel: [-0.05 ("y") -0.025 ("y") 0.025 ("y") 0.05 ("y")] -> w971
                    frame 0, Default {
                    }
                    frame 1 {
                    }
                    frame 2 {
                    }
                    frame 3 {
                    }
                  }
                }
                "Sigma" <- w969
                n492 = Add(x=w967, y=w969) -> (x+y=w968:dbl[])
                "Last Zernike" <- w967
              }
            }
            n493 = In Range and Coerce(upper limit=1.0 ("y"), x=w940, lower limit=-1.0 ("y")) -> (coerced(x)=w931:dbl[])  [unwired: 1 out]
            n494 = Boolean To (0,1)(Boolean="Zernike Enable") -> (0, 1=w929:i16[])
            n495 = Multiply(x=w931, y=w929) -> (x*y=w928:dbl[])
            n496 = call "TLDFMX Calculate Zernike Pattern.vi"("error in (no error)"=w926, "Zernike Amplitudes"=w928, "Zernikes"=u32 4294967295, "instrument handle"=w927) -> ("error out"=w945:errorcluster, "Mirror Pattern"=w946:dbl[], "instrument handle out"=w947:refnum<visa-resource-name>)  [unwired: 5 in]
            n497 = call "TLDFM Set Segment Voltages.vi"("error in (no error)"=w945, "Segment Voltages"=w946, "instrument handle"=w947) -> ("error out"=w936:errorcluster, "instrument handle out"=w944:refnum<visa-resource-name>)  [unwired: 7 in]
            n498 = property on="Fast Scan" class="Bool (strict)"(error in=w936, "Val(Sgnl)"=w937) -> (error out=w938:errorcluster)  [unwired: 1 in, 1 out]
            n499 = property on="SPGD" class="Bool (strict)"(error in=w938, "Val(Sgnl)"=w937) -> (error out=w935:errorcluster)  [unwired: 1 in, 1 out]
            n500 = local write "Zernike Array"(w928) -> ()
          }
          frame True {
            w980 = FALSE ("2D Time-Lapse Measure")
            n501 = local write "Fast Scan Progress"(0.0 ("Fast Scan Progress")) -> ()
            n502 = local write "Fast Scan"(w980) -> ()
            n503 = local write "Current Iteration"(sgl 0.0 ("Current Step")) -> ()
            n504 = local write "SPGD"(w980) -> ()
            n505 = local write "Stop Fast Scan"(w980) -> ()
            n506 = local write "Stop AO Algorithm"(w980) -> ()
          }
        }
      }
      event "Export Z Calibration": Value Change {
        n507 = event-data() -> ()  [unwired: 1 in, 1 out]
        n508 = local read "Z Direction"() -> (w991:bool)
        n509 = local read "Current Iteration"() -> (w989:sgl)
        n510 = Less Or Equal?(x=w989, y=sgl 1.0) -> (x <= y?=w990:bool)
        n511 = Compound Arithmetic op=OR(w991, w990) -> (w992:bool)
        n512 = case shown="False" w992 {
          tunnel: w993 -> [w1006 w1031]
          tunnel: [w1005 w1031] -> w986
          frame False {
            n513 = local read "Current Z Idx"() -> (w1004:i32)
            n514 = Add(x=w1004, y=3) -> (x+y=w1023:i32)
            n515 = Number To Decimal String(number=w1023) -> (decimal integer string=w1024:string)  [unwired: 1 in]
            n516 = Current VI's Path() -> (path=w1020:path)
            n517 = Concatenate Strings("Zernike Calibration_" ("string"), "Note") -> (w1002:string)
            n518 = Strip Path(path=w1020) -> (stripped path=w1021:path)  [unwired: 1 out]
            n519 = Build Path(base path=w1021, name or relative path=w1002) -> (appended path=w1014:path)
            n520 = call <vilib>:"Check if File or Folder Exists.vi"("error in (no error)"=w1006, "path"=w1014) -> ("error out"=w1016:errorcluster, "file or folder exists?"=w1017:bool, "dup path"=w1015:path)  [unwired: 7 in]
            n521 = case shown="False" w1017 {
              tunnel: w1016 -> [w1028 w1029]
              tunnel: [w1027 w1029] -> w1013
              tunnel: [w1026 w1030] -> w1019
              tunnel: w1015 -> [w1025 w1030]
              frame False {
                n522 = Create Folder(path (use dialog)=w1025, error in=w1028) -> (created path=w1026:path, error out=w1027:errorcluster)  [unwired: 1 in, 1 out]
              }
              frame True {
              }
            }
            n523 = property on="Metric Calibration" class="WFChart (strict)"(error in=w1013) -> (error out=w1010:errorcluster, "History Data"=w1012:dbl[][])  [unwired: 1 in, 1 out]
            n524 = Transpose 2D Array(2D array=w1012) -> (transposed array=w1011:dbl[][])
            n525 = call "Save2CSV.vi"("Time Stamp?"=FALSE, "File Name"="Z" ("string"), "error in"=w1010, "Data Name"=w1024, "Data 2D Array"=w1011, "Parent Directory"=w1019) -> ("error out"=w1007:errorcluster)  [unwired: 4 in, 1 out]
            n526 = property on="Metric Calibration" class="WFChart (strict)"(error in=w1007, "History Data"=dbl[][] []) -> (error out=w1005:errorcluster)  [unwired: 1 in, 1 out]
          }
          frame True {
          }
        }
        n527 = while {
          tunnel: [w1098] -> w987
          tunnel: [w1100] -> w999
          tunnel: w986 -> [w1096]
          tunnel: [w1096] -> w985
          stop <- w1101 stop-if-true
          n528 = local read "Zernike Enable"() -> (w1099:bool[])
          n529 = local read "Current Z Idx"() -> (w1097:i32)
          n530 = Index Array(array=w1099, index=w1097) -> (element=w1104:bool)
          n531 = Array Size(array=w1099) -> (size(s)=w1103:i32)
          n532 = case shown="False" w1104 {
            tunnel: w1097 -> [w1107 w1109]
            tunnel: [w1106 w1109] -> w1098
            tunnel: [FALSE ("2D Time-Lapse Measure") TRUE ("2D Time-Lapse Measure")] -> w1102
            frame False {
              n533 = Increment(x=w1107) -> (x+1=w1106:i32)
            }
            frame True {
            }
          }
          n534 = Greater Or Equal?(x=w1098, y=w1103) -> (x >= y?=w1100:bool)
          n535 = local write "Current Z Idx"(w1098) -> ()
          n536 = Compound Arithmetic op=OR(w1102, w1100) -> (w1101:bool)
        }
        n537 = local read "Stop AO Algorithm"() -> (w998:bool)
        n538 = Compound Arithmetic op=OR(w999, w998) -> (w1000:bool)
        n539 = case shown="False" w1000 {
          tunnel: w989 -> [w1055 _]
          tunnel: w994 -> [w1049 w1090]
          tunnel: w985 -> [w1034 w1089]
          tunnel: w987 -> [w1048 _]
          tunnel: [w1041 w1089] -> w996
          tunnel: [w1039 w1090] -> w995
          frame False {
            w1040 = TRUE ("Value (Signaling)")
            n540 = Equal To 0?(x=w1055) -> (x = 0?=w1054:bool)
            n541 = case shown="False" w1054 {
              tunnel: [w1067 dbl[] [0.0, 0.0, 0.0, 0.0, 0.0, 0.0, 0.0, 0.0, 0.0, 0.0, 0.0, 0.0] ("Zernike Array")] -> w1045
              tunnel: w1048 -> [w1059 _]
              tunnel: [w1061 w1086] -> w1036
              tunnel: [w1057 w1086] -> w1032
              tunnel: w1034 -> [w1058 w1084]
              tunnel: [w1058 w1083] -> w1033
              frame False {
                n542 = local read "Zernike Array"() -> (w1069:dbl[])
                n543 = local read "Z Direction"() -> (w1065:bool)
                n544 = local read "Metric Value"() -> (w1062:dbl)
                n545 = Index Array(array=w1069, index=w1059) -> (element=w1068:dbl)
                n546 = case shown="True" w1065 {
                  tunnel: w1068 -> [_ w1074]
                  tunnel: [-1.0 w1076] -> w1063
                  tunnel: w1062 -> [_ w1075]
                  tunnel: [nan ("Metric Value") w1075] -> w1061
                  tunnel: [nan ("Z4: Ast45") w1074] -> w1057
                  frame False {
                    n547 = local write "Z Direction"(TRUE ("Zernike Dir")) -> ()
                  }
                  frame True {
                    n548 = Add(x=w1074, y="Z Cali Step") -> (x+y=w1076:dbl)
                  }
                }
                n549 = Greater?(x=w1063, y=1.0) -> (0:w1066:bool)
                n550 = case shown="True" w1066 {
                  tunnel: w1059 -> [_ w1081]
                  tunnel: w1063 -> [w1078 _]
                  tunnel: [w1078 0.0] -> w1060
                  frame False {
                  }
                  frame True {
                    n551 = Increment(x=w1081) -> (x+1=w1082:i32)
                    n552 = local write "Current Z Idx"(w1082) -> ()
                    n553 = local write "Z Direction"(FALSE ("Zernike Dir")) -> ()
                  }
                }
                n554 = Replace Array Subset(array=w1069, new element=w1060, index=w1059) -> (w1067:dbl[])
              }
              frame True {
                w1086 = nan ("Metric Value")
                n555 = local write "Z Direction"(FALSE ("Zernike Dir")) -> ()
                n556 = property on="Metric Calibration" class="WFChart (strict)"(error in=w1084, "History Data"=dbl[][] []) -> (error out=w1083:errorcluster)  [unwired: 1 in, 1 out]
              }
            }
            n557 = Increment(x=w1055) -> (x+1=w1056:sgl)
            n558 = local write "Current Iteration"(w1056) -> ()
            n559 = In Range and Coerce(upper limit=1.0 ("y"), x=w1045, lower limit=-1.0 ("y")) -> (coerced(x)=w1044:dbl[])  [unwired: 1 out]
            n560 = call "TLDFMX Calculate Zernike Pattern.vi"("error in (no error)"=w1033, "Zernike Amplitudes"=w1044, "Zernikes"=u32 4294967295, "instrument handle"=w1049) -> ("error out"=w1050:errorcluster, "Mirror Pattern"=w1051:dbl[], "instrument handle out"=w1052:refnum<visa-resource-name>)  [unwired: 5 in]
            n561 = call "TLDFM Set Segment Voltages.vi"("error in (no error)"=w1050, "Segment Voltages"=w1051, "instrument handle"=w1052) -> ("error out"=w1043:errorcluster, "instrument handle out"=w1039:refnum<visa-resource-name>)  [unwired: 7 in]
            n562 = property on="Fast Scan" class="Bool (strict)"(error in=w1043, "Val(Sgnl)"=w1040) -> (error out=w1042:errorcluster)  [unwired: 1 in, 1 out]
            n563 = property on="Export Z Calibration" class="Bool (strict)"(error in=w1042, "Val(Sgnl)"=w1040) -> (error out=w1041:errorcluster)  [unwired: 1 in, 1 out]
            n564 = Build Array(w1032) -> (w1037:dbl[])
            n565 = Build Array(w1036) -> (w1035:dbl[])
            n566 = local write "Zernike Array"(w1044) -> ()
            n567 = Build Array(w1037, w1035) -> (→"Metric Calibration":dbl[][])
          }
          frame True {
            w1091 = FALSE ("2D Time-Lapse Measure")
            n568 = local write "Export Z Calibration"(w1091) -> ()
            n569 = local write "Current Iteration"(sgl 0.0 ("Current Step")) -> ()
            n570 = local write "Z Direction"(FALSE ("Zernike Dir")) -> ()
            n571 = local write "Fast Scan Progress"(0.0 ("Fast Scan Progress")) -> ()
            n572 = local write "Current Z Idx"(0 ("Curr Zernike Idx")) -> ()
            n573 = local write "Fast Scan"(w1091) -> ()
            n574 = local write "Stop Fast Scan"(w1091) -> ()
            n575 = local write "Stop AO Algorithm"(w1091) -> ()
          }
        }
      }
      event "Measure": Value Change {
        n576 = event-data() -> ()  [unwired: 1 in, 1 out]
        n577 = flat-sequence {
          tunnel: w1132 -> [w1137]
          tunnel: [w1137] -> w1131
          tunnel: [w1136] -> w1129
          tunnel: [w1135] -> w1127
          tunnel: w1126 -> [w1135]
          tunnel: [w1134] -> w1125
          tunnel: w1124 -> [w1134]
          tunnel: w1121 -> [w1133]
          tunnel: [w1133] -> w1120
          tunnel: w1131 -> [w1172]
          tunnel: [w1172] -> w1130
          tunnel: w1129 -> [w1147]
          tunnel: [w1147] -> w1128
          tunnel: w1127 -> [w1169]
          tunnel: w1125 -> [w1165]
          tunnel: [w1164] -> w1122
          tunnel: w1120 -> [w1159]
          tunnel: [w1152] -> w1116
          tunnel: [w1146] -> w1114
          tunnel: [w1143] -> w1113
          tunnel: [w1142] -> w1112
          tunnel: w1130 -> [w1241]
          tunnel: w1128 -> [w1240]
          tunnel: w1122 -> [w1238]
          tunnel: [w1241] -> w1119
          tunnel: [w1234] -> w1118
          tunnel: w1116 -> [w1239]
          tunnel: [w1240] -> w1115
          tunnel: w1114 -> [w1237]
          tunnel: w1113 -> [w1236]
          tunnel: w1112 -> [w1235]
          tunnel: [w1296] -> w1123
          tunnel: [w1298] -> w1117
          tunnel: w1119 -> [w1298]
          tunnel: w1118 -> [w1296]
          tunnel: w1115 -> [w1292]
          frame #0 {
            n578 = Tick Count (ms)() -> (millisecond timer value=w1136:u32)
          }
          frame #1 {
            w1170 = T13."Measurement" ("Main Tab")
            n579 = local read "AIStartTrigger"() -> (w1139:tag)
            n580 = local read "Calibrated Bias (V)"() -> (w1153:dbl[])
            n581 = local read "AOStartTrigger"() -> (w1138:tag)
            n582 = call "ScanXY.vi"("Scan/Meas Parameters"="Measurement Parameters") -> ("XYcoordinates"=w1156:dbl[][])  [unwired: 10 in]
            n583 = Unbundle By Name("Measurement Parameters") -> ("Pixel Size"=w1162:dbl)
            n584 = case shown="True" "Single Pixel Measure?" {
              tunnel: [w1173 w1174] -> w1155
              tunnel: w1156 -> [w1173 w1175]
              frame False {
              }
              frame True {
                n585 = Multiply(x=w1175, y=0.0) -> (x*y=w1174:dbl[][])
              }
            }
            n586 = call "DAQInit.vi"("AOStartTrigger"=w1138, "AIStartTrigger"=w1139, "Scan/Meas Parameters"="Measurement Parameters", "error in"=w1159, "Functions"=w1170, "Global Parameters"=w1165, "DAQ Channels"=w1169) -> ("error out"=w1160:errorcluster, "Expected Time (s)"=→"Expected Frame Time (s)":dbl, "Tasks Out"=w1171:T14)  [unwired: 2 in]
            n587 = To Long Integer(number=w1162) -> (32bit integer=w1161:i32)
            n588 = while {
              tunnel: w1171 -> [w1225]
              tunnel: w1170 -> [w1194]
              tunnel: w1160 -> [w1184]
              tunnel: w1155 -> [w1224]
              tunnel: w1153 -> [w1223]
              tunnel: w1165 -> [w1192]
              tunnel: "Measurement Parameters" -> [w1193]
              tunnel: [w1221] -> w1168
              tunnel: [w1194] -> w1167
              tunnel: [w1188] -> w1166
              tunnel: [w1199] -> w1164
              tunnel: w1161 -> [w1199]
              tunnel: "# of Frames to Average" -> [w1212]
              tunnel: [w1182] -> w1151
              tunnel: [w1181] -> w1150
              tunnel: [w1180] -> w1149
              tunnel: [w1179] -> w1148
              tunnel: [w1178] -> w1146
              i -> [w1210]
              stop <- w1219 stop-if-true
              n589 = local read "Shutter"() -> (w1185:bool)
              n590 = To Unsigned Long Integer(number=w1210) -> (unsigned 32bit integer=w1198:u32)
              n591 = case shown="False" w1185 {
                tunnel: w1184 -> [w1230 w1232]
                tunnel: [w1229 w1232] -> w1183
                frame False {
                  n592 = local read "Shutter Line"() -> (w1227:tag)
                  n593 = call "ShutterControl.vi"("error in"=w1230, "Shutter Line"=w1227, "Shutter"=TRUE) -> ("error out"=w1229:errorcluster, "Status Indicator"=w1228:bool)  [unwired: 7 in]
                  n594 = local write "Shutter"(w1228) -> ()
                }
                frame True {
                }
              }
              n595 = call "ImageFrame.vi"("Tasks In"=w1225, "Vphases"=w1223, "Functions"=w1194, "error in"=w1183, "XYcoordinates"=w1224) -> ("Tasks Out"=w1221:T14, "Mixer AI Channels Data"=w1222:dbl[][], "DC AI Channel Date"=w1191:dbl[], "error out"=w1187:errorcluster)  [unwired: 6 in, 1 out]
              n596 = Unbundle By Name(w1187) -> ("status"=w1220:bool)
              n597 = Increment(x=w1198) -> (x+1=w1197:u32)
              n598 = call "Analysis.vi"("Functions"=w1194, "error in"=w1187, "Scan/Meas Parameters"=w1193, "Global Parameters"=w1192, "DC AI Channel Data"=w1191, "Mixer AI Channels Data"=w1222) -> ("AI Mix4 Data"=w1207:dbl[], "AI Mix3 Data"=w1204:dbl[], "AI Mix2 Data"=w1202:dbl[], "AI Mix1 Data"=w1200:dbl[], "AI DC Data"=w1218:dbl[], "error out"=w1186:errorcluster)